vi "Main.vi"() -> ()   [LabVIEW 2018] (continued)
"CON2.Toe_E2", "CON2.Toe_E3", "CON2.Toe_E4", "CON2.Toe_E5", "CON2.Toe_E6", "CON2.Toe_E7", "CON2.Toe_E8", "CON2.Toe_E9", "CON2.Toe_E10", "CON2.Toe_F1", "CON2.Toe_F2", "CON2.Toe_F3", "CON2.Toe_F4", "CON2.Toe_F5", "CON2.Toe_F6", "CON2.Toe_F7", "CON2.Toe_F8", "CON2.Toe_F9", "CON2.Toe_F10", "CON2.Toe_F11", "CON2.Toe_G1", "CON2.Toe_G2", "CON2.Toe_G3", "CON2.Toe_G4", "CON2.Toe_G5", "CON2.Toe_G6", "CON2.Toe_G7", "CON2.Toe_G8", "CON2.Toe_G9", "CON2.Toe_G10", "CON2.Toe_G11", "CON2.Toe_H1", "CON2.Toe_H2", "CON2.Toe_H3", "CON2.Toe_H4", "CON2.Toe_H5", "CON2.Toe_H6", "CON2.Toe_H7", "CON2.Toe_H8", "CON2.Toe_H9", "CON2.Toe_H10", "CON2.Toe_H11", "CON2.Toe_J1", "CON2.Toe_J2", "CON2.Toe_J3", "CON2.Toe_J4", "CON2.Toe_J5", "CON2.Toe_J6", "CON2.Toe_J7", "CON2.Toe_J8", "CON2.Toe_J9", "CON2.Toe_J10", "CON2.Toe_J11", "CON2.Toe_K11", "CON4.Toe_A1", "CON4.Toe_A2", "CON4.Toe_A3", "CON4.Toe_A4", "CON4.Toe_A5", "CON4.Toe_A6", "CON4.Toe_A7", "CON4.Toe_A8", "CON4.Toe_A9", "CON4.Toe_A10", "CON4.Toe_B1", "CON4.Toe_B2", "CON4.Toe_B3", "CON4.Toe_B4", "CON4.Toe_B5", "CON4.Toe_B6", "CON4.Toe_B7", "CON4.Toe_B8", "CON4.Toe_B9", "CON4.Toe_B10", "CON4.Toe_C1", "CON4.Toe_C2", "CON4.Toe_C3", "CON4.Toe_C4", "CON4.Toe_C5", "CON4.Toe_C6", "CON4.Toe_C7", "CON4.Toe_C8", "CON4.Toe_C9", "CON4.Toe_C10", "CON4.Toe_D1", "CON4.Toe_D2", "CON4.Toe_D3", "CON4.Toe_D4", "CON4.Toe_D5", "CON4.Toe_D6", "CON4.Toe_D7", "CON4.Toe_D8", "CON4.Toe_D9", "CON4.Toe_D10", "CON4.Toe_E1", "CON4.Toe_E2", "CON4.Toe_E3", "CON4.Toe_E4", "CON4.Toe_E5", "CON4.Toe_E6", "CON4.Toe_E7", "CON4.Toe_E8", "CON4.Toe_E9", "CON4.Toe_E10", "CON4.Toe_F1", "CON4.Toe_F2", "CON4.Toe_F3", "CON4.Toe_F4", "CON4.Toe_F5", "CON4.Toe_F6", "CON4.Toe_F7", "CON4.Toe_F8", "CON4.Toe_F9", "CON4.Toe_F10", "CON4.Toe_F11", "CON4.Toe_G1", "CON4.Toe_G2", "CON4.Toe_G3", "CON4.Toe_G4", "CON4.Toe_G5", "CON4.Toe_G6", "CON4.Toe_G7", "CON4.Toe_G8", "CON4.Toe_G9", "CON4.Toe_G10", "CON4.Toe_G11", "CON4.Toe_H1", "CON4.Toe_H2", "CON4.Toe_H3", "CON4.Toe_H4", "CON4.Toe_H5", "CON4.Toe_H6", "CON4.Toe_H7", "CON4.Toe_H8", "CON4.Toe_H9", "CON4.Toe_H10", "CON4.Toe_H11", "CON4.Toe_J1", "CON4.Toe_J2", "CON4.Toe_J3", "CON4.Toe_J4", "CON4.Toe_J5", "CON4.Toe_J6", "CON4.Toe_J7", "CON4.Toe_J8", "CON4.Toe_J9", "CON4.Toe_J10", "CON4.Toe_J11", "CON4.Toe_K11", "CON1.Toe_A1", "CON1.Toe_A2", "CON1.Toe_A3", "CON1.Toe_A4", "CON1.Toe_A5", "CON1.Toe_A6", "CON1.Toe_A7", "CON1.Toe_A8", "CON1.Toe_A9", "CON1.Toe_A10", "CON1.Toe_B1", "CON1.Toe_B2", "CON1.Toe_B3", "CON1.Toe_B4", "CON1.Toe_B5", "CON1.Toe_B6", "CON1.Toe_B7", "CON1.Toe_B8", "CON1.Toe_B9", "CON1.Toe_B10", "CON1.Toe_C1", "CON1.Toe_C2", "CON1.Toe_C3", "CON1.Toe_C4", "CON1.Toe_C5", "CON1.Toe_C6", "CON1.Toe_C7", "CON1.Toe_C8", "CON1.Toe_C9", "CON1.Toe_C10", "CON1.Toe_D1", "CON1.Toe_D2", "CON1.Toe_D3", "CON1.Toe_D4", "CON1.Toe_D5", "CON1.Toe_D6", "CON1.Toe_D7", "CON1.Toe_D8", "CON1.Toe_D9", "CON1.Toe_D10", "CON1.Toe_E1", "CON1.Toe_E2", "CON1.Toe_E3", "CON1.Toe_E4", "CON1.Toe_E5", "CON1.Toe_E6", "CON1.Toe_E7", "CON1.Toe_E8", "CON1.Toe_E9", "CON1.Toe_E10", "CON1.Toe_F1", "CON1.Toe_F2", "CON1.Toe_F3", "CON1.Toe_F4", "CON1.Toe_F5", "CON1.Toe_F6", "CON1.Toe_F7", "CON1.Toe_F8", "CON1.Toe_F9", "CON1.Toe_F10", "CON1.Toe_F11", "CON1.Toe_G1", "CON1.Toe_G2", "CON1.Toe_G3", "CON1.Toe_G4", "CON1.Toe_G5", "CON1.Toe_G6", "CON1.Toe_G7", "CON1.Toe_G8", "CON1.Toe_G9", "CON1.Toe_G10", "CON1.Toe_G11", "CON1.Toe_H1", "CON1.Toe_H2", "CON1.Toe_H3", "CON1.Toe_H4", "CON1.Toe_H5", "CON1.Toe_H6", "CON1.Toe_H7", "CON1.Toe_H8", "CON1.Toe_H9", "CON1.Toe_H10", "CON1.Toe_H11", "CON1.Toe_J1", "CON1.Toe_J2", "CON1.Toe_J3", "CON1.Toe_J4", "CON1.Toe_J5", "CON1.Toe_J6", "CON1.Toe_J7", "CON1.Toe_J8", "CON1.Toe_J9", "CON1.Toe_J10", "CON1.Toe_J11", "CON1.Toe_K11", "C196.Toe_01", "C196.Toe_02", "CON10", "CON10.Toe_01", "CON10.Toe_02", "CON10.Toe_03", "CON10.Toe_04", "CON10.Toe_05", "CON9", "CON9.Toe_01", "CON9.Toe_02", "CON9.Toe_03", "CON9.Toe_04", "CON9.Toe_05", "CON9.Toe_06", "CON9.Toe_07", "CON9.Toe_08", "CON9.Toe_09", "CON9.Toe_10", "CON9.Toe_11", "CON9.Toe_12", "CON9.Toe_13", "CON9.Toe_14", "CON9.Toe_15", "CON9.Toe_16", "CON9.Toe_17", "CON9.Toe_18", "CON9.Toe_19", "CON9.Toe_20", "F2", "F2.Toe_01", "F2.Toe_02", "FB5", "FB5.Toe_01", "FB5.Toe_02", "J4", "J4.Toe_01", "J4.Toe_02", "J4.Toe_03", "J4.Toe_04", "J4.Toe_05", "R252.Toe_01", "R252.Toe_02", "R182.Toe_01", "R182.Toe_02", "R310.Toe_01", "R310.Toe_02", "R311.Toe_01", "R311.Toe_02", "R328.Toe_01", "R328.Toe_02", "R75.Toe_01", "R75.Toe_02", "R102.Toe_01", "R102.Toe_02", "U38", "U38.Toe_01", "U38.Toe_02", "U38.Toe_03", "U38.Toe_04", "U38.Toe_05", "U38.Toe_06", "U38.Toe_07", "U38.Toe_08", "U37", "U37.Toe_01", "U37.Toe_02", "U37.Toe_03", "U37.Toe_04", "U37.Toe_05", "U37.Toe_06", "U37.Toe_07", "U37.Toe_08", "U12", "U12.Toe_01", "U12.Toe_02", "U12.Toe_03", "U12.Toe_04", "U12.Toe_05", "U12.Toe_06", "U12.Toe_07", "U12.Toe_08", "U12.Toe_09", "U12.Toe_10", "U12.Toe_11", "U12.Toe_12", "U12.Toe_13", "U12.Toe_14", "U12.Toe_15", "U12.Toe_16", "U6", "U6.Toe_01", "U6.Toe_02", "U6.Toe_03", "U6.Toe_04", "U6.Toe_05", "U6.Toe_06", "U6.Toe_07", "U6.Toe_08", "U6.Toe_09", "U6.Toe_10", "U6.Toe_11", "U6.Toe_12", "U6.Toe_13", "U6.Toe_14", "U6.Toe_15", "U6.Toe_16", "U39", "U39.Toe_01", "U39.Toe_02", "U39.Toe_03", "U39.Toe_04", "U39.Toe_05", "U39.Toe_06", "U31", "U31.Toe_01", "U31.Toe_02", "U31.Toe_03", "U11.Toe_01", "U11.Toe_02", "U11.Toe_03", "U11.Toe_04", "U11.Toe_05", "U11.Toe_06", "U11.Toe_07", "U11.Toe_08", "U11.Toe_09", "U3", "U3.Toe_01", "U3.Toe_02", "U3.Toe_03", "U3.Toe_04", "U3.Toe_05", "U3.Toe_06", "U3.Toe_07", "U3.Toe_08", "U7", "U7.Toe_01", "U7.Toe_02", "U7.Toe_03", "U7.Toe_04", "U7.Toe_05", "U7.Toe_06", "U7.Toe_07", "U7.Toe_08", "U13", "U13.Toe_01", "U13.Toe_02", "U13.Toe_03", "U13.Toe_04", "U13.Toe_05", "U13.Toe_06", "U13.Toe_07", "U13.Toe_08", "U13.Toe_09", "U13.Toe_10", "U13.Toe_11", "U13.Toe_12", "U13.Toe_13", "U13.Toe_14", "U13.Toe_15", "U13.Toe_16", "U13.Toe_17", "U13.Toe_18", "U13.Toe_19", "U13.Toe_20", "U13.Toe_21", "U13.Toe_22", "U13.Toe_23", "U13.Toe_24", "U13.Toe_25", "U13.Toe_26", "U13.Toe_27", "U13.Toe_28", "U13.Toe_29", "U13.Toe_30", "U13.Toe_31", "U13.Toe_32", "U13.Toe_33", "U13.Toe_34", "U13.Toe_35", "U13.Toe_36", "U13.Toe_37", "U13.Toe_38", "U13.Toe_39", "U13.Toe_40", "U13.Toe_41", "U13.Toe_42", "U13.Toe_43", "U13.Toe_44", "U13.Toe_45", "U13.Toe_46", "U13.Toe_47", "U13.Toe_48", "U13.Toe_49", "U13.Toe_50", "U13.Toe_51", "U13.Toe_52", "U13.Toe_53", "U13.Toe_54", "U13.Toe_55", "U13.Toe_56", "U13.Toe_57", "U13.Toe_58", "U13.Toe_59", "U13.Toe_60", "U13.Toe_61", "U13.Toe_62", "U13.Toe_63", "U13.Toe_64", "U13.Toe_65", "U13.Toe_66", "U13.Toe_67", "U13.Toe_68", "U13.Toe_69", "U13.Toe_70", "U13.Toe_71", "U13.Toe_72", "U13.Toe_73", "U13.Toe_74", "U13.Toe_75", "U13.Toe_76", "U13.Toe_77", "U13.Toe_78", "U13.Toe_79", "U13.Toe_80", "U13.Toe_81", "U13.Toe_82", "U13.Toe_83", "U13.Toe_84", "U13.Toe_85", "U13.Toe_86", "U13.Toe_87", "U13.Toe_88", "U13.Toe_89", "U13.Toe_90", "U13.Toe_91", "U13.Toe_92", "U13.Toe_93", "U13.Toe_94", "U13.Toe_95", "U13.Toe_96", "U13.Toe_97", "U13.Toe_98", "U13.Toe_99", "U13.Toe_100", "U13.Toe_101", "U13.Toe_102", "U13.Toe_103", "U13.Toe_104", "U13.Toe_105", "U13.Toe_106", "U13.Toe_107", "U13.Toe_108", "U13.Toe_109", "U13.Toe_110", "U13.Toe_111", "U13.Toe_112", "U13.Toe_113", "U13.Toe_114", "U13.Toe_115", "U13.Toe_116", "U13.Toe_117", "U13.Toe_118", "U13.Toe_119", "U13.Toe_120", "U13.Toe_121", "U13.Toe_122", "U13.Toe_123", "U13.Toe_124", "U13.Toe_125", "U13.Toe_126", "U13.Toe_127", "U13.Toe_128", "U13.Toe_129", "U13.Toe_130", "U13.Toe_131", "U13.Toe_132", "U13.Toe_133", "U13.Toe_134", "U13.Toe_135", "U13.Toe_136", "U13.Toe_137", "U13.Toe_138", "U13.Toe_139", "U13.Toe_140", "U13.Toe_141", "U13.Toe_142", "U13.Toe_143", "U13.Toe_144", "U13.Toe_145", "U13.Toe_146", "U13.Toe_147", "U13.Toe_148", "U13.Toe_149", "U13.Toe_150", "U13.Toe_151", "U13.Toe_152", "U13.Toe_153", "U13.Toe_154", "U13.Toe_155", "U13.Toe_156", "U13.Toe_157", "U13.Toe_158", "U13.Toe_159", "U13.Toe_160", "U13.Toe_161", "U13.Toe_162", "U13.Toe_163", "U13.Toe_164", "U13.Toe_165", "U13.Toe_166", "U13.Toe_167", "U13.Toe_168", "U13.Toe_169", "U13.Toe_170", "U13.Toe_171", "U13.Toe_172", "U13.Toe_173", "U13.Toe_174", "U13.Toe_175", "U13.Toe_176", "U22", "U22.Toe_01", "U22.Toe_02", "U22.Toe_03", "U22.Toe_04", "SW1", "SW1.Toe_01", "SW1.Toe_02", "SW1.Toe_03", "SW1.Toe_04", "SW1.Toe_05", "Q5", "Q5.Toe_01", "Q5.Toe_02", "Q5.Toe_03", "Q4", "Q4.Toe_01", "Q4.Toe_02", "Q4.Toe_03", "Q3", "Q3.Toe_01", "Q3.Toe_02", "Q3.Toe_03", "Q1", "Q1.Toe_01", "Q1.Toe_02", "Q1.Toe_03", "Q2", "Q2.Toe_01", "Q2.Toe_02", "Q2.Toe_03", "CON3.Toe_A1", "CON3.Toe_A2", "CON3.Toe_A3", "CON3.Toe_A4", "CON3.Toe_A5", "CON3.Toe_A6", "CON3.Toe_A7", "CON3.Toe_A8", "CON3.Toe_A9", "CON3.Toe_A10", "CON3.Toe_B1", "CON3.Toe_B2", "CON3.Toe_B3", "CON3.Toe_B4", "CON3.Toe_B5", "CON3.Toe_B6", "CON3.Toe_B7", "CON3.Toe_B8", "CON3.Toe_B9", "CON3.Toe_B10", "CON3.Toe_C1", "CON3.Toe_C2", "CON3.Toe_C3", "CON3.Toe_C4", "CON3.Toe_C5", "CON3.Toe_C6", "CON3.Toe_C7", "CON3.Toe_C8", "CON3.Toe_C9", "CON3.Toe_C10", "CON3.Toe_D1", "CON3.Toe_D2", "CON3.Toe_D3", "CON3.Toe_D4", "CON3.Toe_D5", "CON3.Toe_D6", "CON3.Toe_D7", "CON3.Toe_D8", "CON3.Toe_D9", "CON3.Toe_D10", "CON3.Toe_E1", "CON3.Toe_E2", "CON3.Toe_E3", "CON3.Toe_E4", "CON3.Toe_E5", "CON3.Toe_E6", "CON3.Toe_E7", "CON3.Toe_E8", "CON3.Toe_E9", "CON3.Toe_E10", "CON3.Toe_F1", "CON3.Toe_F2", "CON3.Toe_F3", "CON3.Toe_F4", "CON3.Toe_F5", "CON3.Toe_F6", "CON3.Toe_F7", "CON3.Toe_F8", "CON3.Toe_F9", "CON3.Toe_F10", "CON3.Toe_F11", "CON3.Toe_G1", "CON3.Toe_G2", "CON3.Toe_G3", "CON3.Toe_G4", "CON3.Toe_G5", "CON3.Toe_G6", "CON3.Toe_G7", "CON3.Toe_G8", "CON3.Toe_G9", "CON3.Toe_G10", "CON3.Toe_G11", "CON3.Toe_H1", "CON3.Toe_H2", "CON3.Toe_H3", "CON3.Toe_H4", "CON3.Toe_H5", "CON3.Toe_H6", "CON3.Toe_H7", "CON3.Toe_H8", "CON3.Toe_H9", "CON3.Toe_H10", "CON3.Toe_H11", "CON3.Toe_J1", "CON3.Toe_J2", "CON3.Toe_J3", "CON3.Toe_J4", "CON3.Toe_J5", "CON3.Toe_J6", "CON3.Toe_J7", "CON3.Toe_J8", "CON3.Toe_J9", "CON3.Toe_J10", "CON3.Toe_J11", "CON3.Toe_K11", "D4", "D4.Toe_0A", "D4.Toe_0C", "D2", "D2.Toe_0A", "D2.Toe_0C", "R7.Toe_01", "R7.Toe_02", "R2.Toe_01", "R2.Toe_02", "R1.Toe_01", "R1.Toe_02", "R21.Toe_01", "R21.Toe_02", "R11.Toe_01", "R11.Toe_02", "R9.Toe_01", "R9.Toe_02", "R13.Toe_01", "R13.Toe_02", "R16.Toe_01", "R16.Toe_02", "R15.Toe_01", "R15.Toe_02", "D3", "D3.Toe_0A", "D3.Toe_0C", "R5.Toe_01", "R5.Toe_02", "R17.Toe_01", "R17.Toe_02", "R10.Toe_01", "R10.Toe_02", "F1", "F1.Toe_01", "F1.Toe_02", "D1", "D1.Toe_0A", "D1.Toe_0C", "BRK1.Toe_NPTH", "BRK1.Toe_NPTH", "BRK1.Toe_NPTH", "BRK9.Toe_NPTH", "BRK9.Toe_NPTH", "BRK9.Toe_NPTH", "BRK11.Toe_NPTH", "BRK11.Toe_NPTH", "BRK11.Toe_NPTH", "BRK10.Toe_NPTH", "BRK10.Toe_NPTH", "BRK10.Toe_NPTH", "BRK7.Toe_NPTH", "BRK7.Toe_NPTH", "BRK7.Toe_NPTH", "BRK8.Toe_NPTH", "BRK8.Toe_NPTH", "BRK8.Toe_NPTH", "BRK12.Toe_NPTH", "BRK12.Toe_NPTH", "BRK12.Toe_NPTH", "BRK2.Toe_NPTH", "BRK2.Toe_NPTH", "BRK2.Toe_NPTH", "BRK6.Toe_NPTH", "BRK6.Toe_NPTH", "BRK6.Toe_NPTH", "U28", "U28.Toe_01", "U28.Toe_02", "U28.Toe_03", "R224.Toe_01", "R224.Toe_02", "R228.Toe_01", "R228.Toe_02", "U29", "U29.Toe_01", "U29.Toe_02", "U29.Toe_03", "U30", "U30.Toe_01", "U30.Toe_02", "U30.Toe_03", "R229.Toe_01", "R229.Toe_02", "CON5", "CON6", "CON7", "CON8"], "Not Fitted position[x][y] "=[[10.358, 24.671], [14.308, 23.996], [12.108, 24.671], [124.31, 151.908], [45.074, 23.638], [29.594, 24.144], [52.458, 23.646], [45.95, 23.6], [43.85, 23.275], [29.594, 22.138], [28.024, 24.188], [161.3, 67.0], [167.067, 95.562], [167.067, 87.942], [167.067, 80.322], [54.1, 40.9], [48.325, 41.91], [38.45, 40.9], [36.375, 41.9], [22.751, 40.9], [20.601, 41.9], [4.982, 40.9], [2.907, 41.9], [22.4, 32.1], [38.497, 32.095], [1.825, 30.1], [4.776, 32.097], [106.967, 147.4], [157.991, 18.914], [153.86, 15.7], [168.825, 6.6], [168.817, 8.5], [112.15, 40.619], [113.95, 40.619], [99.042, 64.701], [147.921, 50.525], [147.925, 51.475], [99.042, 86.148], [146.3, 27.925], [147.85, 30.222], [98.542, 109.395], [144.15, 23.5], [145.1, 23.5], [160.017, 185.425], [131.917, 173.425], [103.817, 185.425], [130.459, 62.033], [143.817, 15.0], [114.5, 28.5], [113.05, 38.072], [152.9, 18.776], [159.762, 18.918], [168.317, 4.153], [152.774, 85.465], [133.508, 61.004], [130.459, 60.283], [75.721, 173.425], [92.366, 174.813], [114.279, 181.485], [114.279, 183.3], [137.49, 164.896], [142.379, 169.485], [142.379, 171.3], [159.66, 169.194], [163.918, 169.24], [163.026, 169.24], [87.298, 176.82], [86.638, 168.917], [86.633, 169.935], [90.0, 192.825], [169.892, 113.0], [169.892, 63.0], [0.175, 63.0], [169.892, 163.0], [0.175, 113.0], [169.892, 13.0], [147.0, 192.825], [0.175, 163.0], [19.425, 30.1], [35.375, 30.1], [50.308, 30.146]], "Not Tested position[x][y]"=array1720x2[3440 elements], "CAD Layers"=[{"1st Filtered Array out"=array[46807 elements], "2nd Filtered Array out"=array[46807 elements]}, {"1st Filtered Array out"=array[492003 elements], "2nd Filtered Array out"=array[492003 elements]}, {"1st Filtered Array out"=array[314618 elements], "2nd Filtered Array out"=array[314618 elements]}, {"1st Filtered Array out"=array[31626 elements], "2nd Filtered Array out"=array[31626 elements]}, {"1st Filtered Array out"=array[569211 elements], "2nd Filtered Array out"=array[569211 elements]}], "Xyz File Exist? "=TRUE, "Options"={"Enable Not Tested Components"=FALSE, "Enable Not Fited Components"=FALSE, "Enable Labels"=FALSE}, "Origin XY Scale Ranges"={"XScale.Max"=0.0, "XScale.Min"=0.0, "YScale.Max"=0.0, "YScale.Min"=0.0}} ("DataOut")
        w105 = "Initial Message" ("Initial Message")
        # "This is a simulation code for Test Coverage Dialog"
        # "Example Data"
        # "Bundle control references and a sample string value."
        # "Initialize - All initialization work should take place in this message, since other loops can potentially enqueue messages that execute immediately after this one."
        n34 = call-poly "Enqueue Message.vi"("error in (no error)"=w113, "Message Data"=w105, "Message"="Update Display", "Message Queue"=w106) -> ("error out"=w88:errorcluster)  [unwired: 6 in, 1 out]
        n35 = control-ref of="XY Graph"() -> (w104:refnum<vi>)
        n36 = property class="XYGraph (strict)"(reference=w104, "Cursor.Visible"=TRUE) -> (reference out=w87:refnum<vi>)  [unwired: 1 in, 1 out]
        n37 = Unbundle By Name(w96) -> ("Not fitted components"=w97:string[], "Not tested components"=w77:string[], "Not Fitted position[x][y]"=w78:dbl[][], "Not Tested position[x][y]"=w79:dbl[][], "CAD Layers"=w80:T8)
        n38 = call "PCB Coverage graph.vi"("UpdatedData"=w96, "error in (no error)"=w88, "XY Graph"=w87, "index"=0, "Disable Autoscale"=FALSE, "Initialise graph"=TRUE) -> ("error out"=w86:errorcluster)  [unwired: 13 in]
        n39 = property class="XYGraph (strict)"(reference=w87, error in=w86) -> (error out=w85:errorcluster, "XScale.Maximum"=w84:dbl, "XScale.Minimum"=w83:dbl, "YScale.Maximum"=w82:dbl, "YScale.Minimum"=w81:dbl)  [unwired: 1 out]
        n40 = control-ref of="Enable Not Tested Components"() -> (w91:refnum<vi>)
        n41 = control-ref of="Enable Not Fited Components"() -> (w90:refnum<vi>)
        n42 = control-ref of="Enable Labels"() -> (w89:refnum<vi>)
        n43 = control-ref of="Reload"() -> (w111:refnum<vi>)
        n44 = control-ref of="Save  to file"() -> (w110:refnum<vi>)
        n45 = control-ref of="Exit Button"() -> (w108:refnum<vi>)
        n46 = control-ref of="Not Tested Components"() -> (w99:refnum<vi>)
        n47 = control-ref of="Not Fitted Components"() -> (w98:refnum<vi>)
        n48 = control-ref of="Event Log"() -> (w109:refnum<vi>)
        n49 = Bundle By Name(cluster=w102, "Do Something Ref"=w111, "Do Something Else Ref"=w110, "Data Display Ref"=w109, "Exit Button Ref"=w108, "String <Replace Me>"=w105, "CAD_Data"=cluster{dbl[], dbl[]}[] [{array[1801 elements], array[1801 elements]}, {array[46807 elements], array[46807 elements]}, {array[492003 elements], array[492003 elements]}, {array[314618 elements], array[314618 elements]}, {array[31626 elements], array[31626 elements]}, {array[569211 elements], array[569211 elements]}] ("Value"), "Reference.XY Graph"=w87, "CAD data Origin.Not fitted components"=w97, "CAD data Origin.Not tested components"=w77, "CAD data Origin.Not Fitted position[x][y]"=w78, "CAD data Origin.Not Tested position[x][y]"=w79, "CAD data Origin.CAD Layers"=w80, "CAD data Origin.Xyz File Exist?"=TRUE ("CAD data.Xyz File Exist?"), "CAD data Origin.Options"=T4 {"Enable Not Tested Components"=TRUE, "Enable Not Fited Components"=TRUE, "Enable Labels"=TRUE} ("CAD data.Options"), "Reference.Not Tested Components"=w99, "Reference.Not Fitted Components"=w98, "Reference.Enable Not Tested Components"=w91, "Reference.Enable Not Fited Components"=w90, "Reference.Enable Labels"=w89, "CAD data Origin.Origin XY Scale Ranges.XScale.Max"=w84, "CAD data Origin.Origin XY Scale Ranges.XScale.Min"=w83, "CAD data Origin.Origin XY Scale Ranges.YScale.Max"=w82, "CAD data Origin.Origin XY Scale Ranges.YScale.Min"=w81) -> (w112:T1)
      }
      frame "Reload" {
        # "Reload CAD layers"
        n50 = call-poly "Enqueue Message.vi"("error in (no error)"=w121, "Message Data"="Reload button pressed" ("\"Do Something\" button pressed"), "Message"="Update Display", "Message Queue"=w119) -> ("error out"=w120:errorcluster, "dup Message Queue"=w116:refnum<queue>)  [unwired: 6 in]
        n51 = call-poly "Enqueue Message.vi"("error in (no error)"=w120, "Message"="Initialize", "Message Queue"=w116) -> ("error out"=w115:errorcluster)  [unwired: 7 in, 1 out]
      }
      frame "Save to file" {
        # "#CodeRecommended -"
        n52 = call-poly "Enqueue Message.vi"("error in (no error)"=w127, "Message Data"="\"Save to file" ("\"Do Something Else\" button pressed"), "Message"="Update Display", "Message Queue"=w125) -> ("error out"=w126:errorcluster)  [unwired: 6 in, 1 out]
        n53 = Merge Errors(w126) -> (w128:errorcluster)
      }
      frame "Update Display" {
        # "#CodeRecommended -"
        # "Update Display - Convert the message data to a string to display in the Data Display indicator."
        n54 = Variant To Data(error in=w134, type="", Variant=w133) -> (data=→"Event Log":string, error out=w131:errorcluster)
        n55 = Merge Errors(w131) -> (w135:errorcluster)
      }
      frame "Error" {
        # "#CodeRecommended - If you ever change the name of this \"Error\" message, you'll need to update the name in the Check Loop Error.vi as well."
        # "#CodeRecommended - Consider creating a system for logging errors in some way. These errors are for notification purposes only. Handling of specific errors should be performed in the message frames that generated the error."
        # "Error - Display an error dialog. This message is sent by the \"Error Handler\" VIs at the end of other loops in this application."
        n56 = Variant To Data(error in=w143, type=errorcluster {"status"=FALSE, "code"=0, "source"=""} ("error constant"), Variant=w141) -> (data=w139:errorcluster, error out=w138:errorcluster)
        n57 = call <vilib>:"Simple Error Handler.vi"("error in (no error)"=w139) -> ()  [unwired: 4 in, 5 out]
        n58 = Merge Errors(w138) -> (w137:errorcluster)
      }
      frame "Confirm Quit" {
        # "#CodeNeeded - If you want to provide an \"Are you sure\" dialog (or some other notification) before the application exits, place that code here. This message is typically sent from a Panel Close? event."
        # "Confirm Quit - Message that can confirm whether or not the user wants to exit the application."
        n59 = call-poly "Enqueue Message.vi"("Priority Message? (F)"=TRUE, "error in (no error)"=w150, "Message"="Exit", "Message Queue"=w146) -> ("error out"=w147:errorcluster)  [unwired: 6 in, 1 out]
        n60 = Merge Errors(w147) -> (w148:errorcluster)
      }
      frame "---Copy This Frame---" {
        # "Duplicate this frame when creating new messages.  Change this comment in the duplicated frame to describe this message."
        n61 = Merge Errors(w153) -> (w151:errorcluster)
      }
      frame "Scale Range Change" {
        (unwired) FALSE
        # "Original ratio"
        # "Whent zoom in/out, keep scale ratio unchanged."
        n62 = Unbundle By Name(w156) -> ("Reference.XY Graph"=w155:refnum<vi>, "CAD data Origin.Origin XY Scale Ranges"=w154:T9)
        n63 = property class="XYGraph (strict)"(reference=w155) -> (reference out=w187:refnum<vi>, error out=w171:errorcluster, "XScale.Maximum"=w176:dbl, "XScale.Minimum"=w175:dbl, "YScale.Maximum"=w178:dbl, "YScale.Minimum"=w177:dbl)  [unwired: 1 in]
        n64 = Unbundle By Name(w154) -> ("XScale.Max"=w186:dbl, "XScale.Min"=w185:dbl, "YScale.Max"=w184:dbl, "YScale.Min"=w183:dbl)
        n65 = Subtract(x=w186, y=w185) -> (x-y=w181:dbl)
        n66 = Subtract(x=w184, y=w183) -> (x-y=w182:dbl)
        n67 = Divide(x=w182, y=w181) -> (x/y=w174:dbl)
        n68 = Subtract(x=w178, y=w177) -> (x-y=w173:dbl)
        n69 = Subtract(x=w176, y=w175) -> (x-y=w172:dbl)
        n70 = Divide(x=w173, y=w172) -> (x/y=w180:dbl)
        n71 = Greater Or Equal?(x=w180, y=w174) -> (x >= y?=w179:bool)
        n72 = case shown="True" w179 {
          tunnel: w178 -> [w214 w234]
          tunnel: [w219 w234] -> w162
          tunnel: [w208 w233] -> w161
          tunnel: w177 -> [w213 w233]
          tunnel: w176 -> [w221 w229]
          tunnel: [w221 w226] -> w164
          tunnel: w175 -> [w220 w228]
          tunnel: [w220 w223] -> w163
          tunnel: w174 -> [w217 w231]
          tunnel: w173 -> [_ w232]
          tunnel: w172 -> [w218 _]
          frame False {
            # "New y/x ratio > origin"
            # "Keep Xscale, match Yscale with the origin"
            n73 = Add(x=w214, y=w213) -> (x+y=w211:dbl)
            n74 = Multiply(x=w217, y=w218) -> (x*y=w216:dbl)
            n75 = Divide(x=w211, y=2.0) -> (x/y=w210:dbl)
            n76 = Divide(x=w216, y=2.0) -> (x/y=w209:dbl)
            n77 = Add(x=w210, y=w209) -> (x+y=w219:dbl)
            n78 = Subtract(x=w210, y=w209) -> (x-y=w208:dbl)
          }
          frame True {
            w222 = 2.0 ("y")
            # "Keep Yscale, match Xscale with the original"
            n79 = Add(x=w229, y=w228) -> (x+y=w227:dbl)
            n80 = Divide(x=w232, y=w231) -> (x/y=w230:dbl)
            n81 = Divide(x=w227, y=w222) -> (x/y=w225:dbl)
            n82 = Divide(x=w230, y=w222) -> (x/y=w224:dbl)
            n83 = Add(x=w225, y=w224) -> (x+y=w226:dbl)
            n84 = Subtract(x=w225, y=w224) -> (x-y=w223:dbl)
          }
        }
        n85 = property class="XYGraph (strict)"(reference=w187, error in=w171, "XScale.Maximum"=w164, "XScale.Minimum"=w163, "YScale.Maximum"=w162, "YScale.Minimum"=w161) -> (reference out=w170:refnum<vi>, error out=w168:errorcluster)
        n86 = property class="XYGraph (strict)"(reference=w170, error in=w168) -> (reference out=w169:refnum<vi>, error out=w167:errorcluster, "Cursor.Cursor X"=w166:dbl, "Cursor.Cursor Y"=w165:dbl)
        n87 = In Range and Coerce(upper limit=w164, x=w166, lower limit=w163) -> (In Range?=w160:bool)  [unwired: 1 out]
        n88 = In Range and Coerce(upper limit=w162, x=w165, lower limit=w161) -> (In Range?=w159:bool)  [unwired: 1 out]
        n89 = And(x=w160, y=w159) -> (x .and. y?=w158:bool)
        n90 = case shown="False" w158 {
          tunnel: w164 -> [w201 _]
          tunnel: w163 -> [w200 _]
          tunnel: w162 -> [w196 _]
          tunnel: w161 -> [w195 _]
          tunnel: [w193 w207] -> w157
          tunnel: w169 -> [w191 _]
          tunnel: w167 -> [w190 w207]
          frame False {
            w192 = 2.0 ("y")
            # "If cursor is invisible, bring it back."
            n91 = Add(x=w201, y=w200) -> (x+y=w199:dbl)
            n92 = Add(x=w196, y=w195) -> (x+y=w197:dbl)
            n93 = Divide(x=w197, y=w192) -> (x/y=w194:dbl)
            n94 = Divide(x=w199, y=w192) -> (x/y=w198:dbl)
            n95 = Bundle By Name(cluster=T5 {"X"=0.0, "Y"=0.0} ("Cursor.Cursor Position"), "X"=w198, "Y"=w194) -> (w203:T5)
            n96 = property class="XYGraph (strict)"(reference=w191, error in=w190, "Cursor.Cursor Index"=0, "Cursor.Cursor Position"=w203, "Cursor.CursorMode"=u32 1 ("Cursor.Cursor Mode"), "ActPaletteTool"=0 ("Palette:Active Tool")) -> (error out=w193:errorcluster)  [unwired: 1 out]
          }
          frame True {
          }
        }
        n97 = Merge Errors(w157, w189) -> (w188:errorcluster)
      }
      frame "Update CAD Layers" {
        w254 = TRUE  # disable autoscale
        # "Duplicate this frame when creating new messages.  Change this comment in the duplicated frame to describe this message."
        n98 = Unbundle By Name(w253) -> ("Reference.XY Graph"=w250:refnum<vi>, "Reference.Enable Not Tested Components"=w249:refnum<vi>, "Reference.Enable Not Fited Components"=w247:refnum<vi>, "Reference.Enable Labels"=w246:refnum<vi>, "CAD data Origin"=w241:T7, "Reference.Not Tested Components"=w243:refnum<vi>, "Reference.Not Fitted Components"=w242:refnum<vi>)
        n99 = control-ref of="This VI"() -> (w252:refnum<vi>)
        n100 = property class="Bool (strict)"(reference=w249) -> ("Value"=w248:bool)  [unwired: 1 in, 2 out]
        n101 = property class="Bool (strict)"(reference=w247) -> ("Value"=w245:bool)  [unwired: 1 in, 2 out]
        n102 = property class="Bool (strict)"(reference=w246) -> ("Value"=w244:bool)  [unwired: 1 in, 2 out]
        n103 = property class="VI"(reference=w252, error in=w251) -> (error out=w265:errorcluster, "Panel"=w266:refnum<vi>)  [unwired: 1 out]
        n104 = Bundle By Name(cluster=w241, "Options.Enable Not Tested Components"=w248, "Options.Enable Not Fited Components"=w245, "Options.Enable Labels"=w244) -> (w257:T7)
        n105 = property class="Pnl"(reference=w266, error in=w265, "DeferPanUpdts"=TRUE ("Defer Panel Updates")) -> (reference out=w261:refnum<vi>, error out=w256:errorcluster)
        n106 = call "Data Update.vi"("UpdatedDataIn"=w257, "OriginData"=w241, "error in (no error)"=w256) -> ("UpdateDataOut"=w239:T7, "error out"=w255:errorcluster)  [unwired: 11 in]
        n107 = Unbundle By Name(w239) -> ("Not fitted components"=w236:string[], "Not tested components"=w237:string[])
        n108 = call "PCB Coverage graph.vi"("UpdatedData"=w239, "error in (no error)"=w255, "XY Graph"=w250, "index"=0, "Disable Autoscale"=w254, "Initialise graph"=TRUE) -> ("error out"=w260:errorcluster)  [unwired: 13 in]
        n109 = Bundle By Name(cluster=w253, "CAD data Update"=w239) -> (w240:T1)
        n110 = property on="Property Node" class="LstBox (strict)"(reference=w243, error in=w260, "Item Names"=w237) -> (error out=w238:errorcluster)  [unwired: 1 out]
        n111 = property on="Property Node" class="LstBox (strict)"(reference=w242, error in=w238, "Item Names"=w236) -> (error out=w262:errorcluster)  [unwired: 1 out]
        n112 = property class="Pnl"(reference=w261, error in=w262, "DeferPanUpdts"=FALSE ("Defer Panel Updates")) -> (error out=w235:errorcluster)  [unwired: 1 out]
        n113 = Merge Errors(w235, w251) -> (w267:errorcluster)
      }
      frame "Mouse Up" {
        w272 = TRUE ("Name Visible")
        # "Mouse Up"